vi "TLB Native Dynamic Events ver 0.26d.vi"() -> ()   [LabVIEW 2018] (continued)
                  tunnel: w1878 -> [w1884 w1890]
                  frame False {
                    n645 = for {
                      tunnel: string[] ["CLOSE CLAW", "START TIMER"] ("element") -> [w1887] mode=indexing
                      shift-right: [w1889] -> w1886
                      shift-left: w1884 -> [w1888]
                      n646 = Enqueue Element(queue=w1888, element=w1887) -> (queue out=w1889:refnum<queue>)  [unwired: 2 in, 2 out]
                    }
                  }
                  frame True {
                    n647 = for {
                      shift-right: [w1894] -> w1892
                      shift-left: w1890 -> [w1895]
                      tunnel: string[] ["READ STEPPER VALUES", "", ""] -> [w1893] mode=indexing
                      n648 = Enqueue Element(queue=w1895, element=w1893) -> (queue out=w1894:refnum<queue>)  [unwired: 2 in, 2 out]
                    }
                  }
                }
                n649 = Or(x=w1877, y=w1873) -> (x .or. y?=w1880:bool)
                n650 = Select(t=State_Type_Definitions,_for_0.26g_versions_and_later_2."True Stop" ("Enum"), s=w1873, f=State_Type_Definitions,_for_0.26g_versions_and_later_2."Task 8K: RAISE MY SWORD" ("Enum")) -> (s? t:f=w1875:T18)
                n651 = Select(t=w1875, s=w1880, f=State_Type_Definitions,_for_0.26g_versions_and_later_2."Task 8J: CLOSE CLAW" ("Enum")) -> (s? t:f=w1879:T18)
              }
              frame "Exit" {
                n652 = for {
                  shift-right: [w1902] -> w1899
                  shift-left: w1896 -> [w1903]
                  tunnel: string[] ["STOP", "RESET ENCODERS", "RESET YAW", "ARDUINO MODE 0"] -> [w1901] mode=indexing
                  n653 = Enqueue Element(queue=w1903, element=w1901) -> (queue out=w1902:refnum<queue>)  [unwired: 2 in, 2 out]
                }
              }
            }
          }
          frame 37 {
            # ">>> yStepper command>>>"
            # ">> Manual override >>"
            n654 = Dequeue Element(queue=w1914, timeout in ms (-1)=w1913, error in (no error)=w1915) -> (element=w1912:T10)  [unwired: 3 out]
            n655 = Equal?(x=w1911, y=u8 60) -> (x = y?=w1909:bool)
            n656 = case shown="\"Start Task 1\", Default" w1912 {
              tunnel: [w1925 State_Type_Definitions,_for_0.26g_versions_and_later_2."True Stop" ("Enum")] -> w1916
              tunnel: [w1928 w1945] -> w1917
              tunnel: [State_Type_Definitions,_for_0.26g_versions_and_later_2."Idle" ("Enum") State_Type_Definitions,_for_0.26g_versions_and_later_2."Shutdown" ("Enum")] -> w1918
              tunnel: w1909 -> [w1924 _]
              tunnel: w1908 -> [w1923 _]
              tunnel: w1907 -> [w1919 w1942]
              frame "Start Task 1", Default {
                # "Stays in Task 5_A until stepper reaches desired \nheight"
                # "T: Go back to idle, F: Continue with task\""
                # ">> Manual override >>"
                n657 = case shown="True" w1924 {
                  tunnel: [w1932 w1938] -> w1928
                  tunnel: w1919 -> [w1930 w1936]
                  frame False {
                    n658 = for {
                      tunnel: string[] ["Z STEPPER CAM HEIGHT", "READ STEPPER VALUES"] ("element") -> [w1933] mode=indexing
                      shift-right: [w1935] -> w1932
                      shift-left: w1930 -> [w1934]
                      n659 = Enqueue Element(queue=w1934, element=w1933) -> (queue out=w1935:refnum<queue>)  [unwired: 2 in, 2 out]
                    }
                  }
                  frame True {
                    n660 = for {
                      shift-right: [w1940] -> w1938
                      shift-left: w1936 -> [w1941]
                      tunnel: string[] ["CAM CLOSE", "DISPOSE CAM BUFFERS", "DISPOSE PROC BUFFERS", "RESET ENCODERS"] -> [w1939] mode=indexing
                      n661 = Enqueue Element(queue=w1941, element=w1939) -> (queue out=w1940:refnum<queue>)  [unwired: 2 in, 2 out]
                    }
                  }
                }
                n662 = Or(x=w1924, y=w1923) -> (x .or. y?=w1926:bool)
                n663 = Select(t=State_Type_Definitions,_for_0.26g_versions_and_later_2."True Stop" ("Enum"), s=w1923, f=State_Type_Definitions,_for_0.26g_versions_and_later_2."True Stop" ("Enum")) -> (s? t:f=w1920:T18)
                n664 = Select(t=w1920, s=w1926, f=State_Type_Definitions,_for_0.26g_versions_and_later_2."Task 8K: RAISE MY SWORD" ("Enum")) -> (s? t:f=w1925:T18)
              }
              frame "Exit" {
                n665 = for {
                  shift-right: [w1948] -> w1945
                  shift-left: w1942 -> [w1949]
                  tunnel: string[] ["STOP", "RESET ENCODERS", "RESET YAW", "ARDUINO MODE 0"] -> [w1947] mode=indexing
                  n666 = Enqueue Element(queue=w1949, element=w1947) -> (queue out=w1948:refnum<queue>)  [unwired: 2 in, 2 out]
                }
              }
            }
          }
          frame 38 {
            # ">>> Motor control cluster >>>"
            # ">> Stepper height reeached >>"
            # ">>> yStepper command>>>"
            # ">> Manual override >>"
            n667 = Dequeue Element(queue=w1961, timeout in ms (-1)=w1956, error in (no error)=w1960) -> (element=w1964:T10)  [unwired: 3 out]
            n668 = Equal?(x=w1958, y=u8 50) -> (x = y?=w1962:bool)
            n669 = case shown="\"Start Task 1\", Default" w1964 {
              tunnel: [w1975 State_Type_Definitions,_for_0.26g_versions_and_later_2."True Stop" ("Enum")] -> w1954
              tunnel: [w1973 w1990] -> w1953
              tunnel: w1957 -> [w1972 _]
              tunnel: w1959 -> [w1966 _]
              tunnel: [State_Type_Definitions,_for_0.26g_versions_and_later_2."Idle" ("Enum") State_Type_Definitions,_for_0.26g_versions_and_later_2."Shutdown" ("Enum")] -> w1955
              tunnel: w1962 -> [w1965 _]
              frame "Start Task 1", Default {
                # ">> WIill proceed to part ii if not manual override >>"
                # ">>If ENABLE or Trigger is set to true>>"
                n670 = Or(x=w1965, y=w1966) -> (x .or. y?=w1967:bool)
                n671 = case shown="False" w1965 {
                  tunnel: [w1978 w1984] -> w1973
                  tunnel: w1972 -> [w1977 w1983]
                  frame False {
                    n672 = for {
                      shift-right: [w1980] -> w1978
                      shift-left: w1977 -> [w1981]
                      tunnel: string[] ["Z STEPPER BOX HEIGHT", "READ STEPPER VALUES"] ("element") -> [w1979] mode=indexing
                      n673 = Enqueue Element(queue=w1981, element=w1979) -> (queue out=w1980:refnum<queue>)  [unwired: 2 in, 2 out]
                    }
                  }
                  frame True {
                    n674 = for {
                      shift-right: [w1986] -> w1984
                      shift-left: w1983 -> [w1987]
                      tunnel: string[] ["READ NAVX", "RESET FLAGS", "", "", "", ""] -> [w1985] mode=indexing
                      n675 = Enqueue Element(queue=w1987, element=w1985) -> (queue out=w1986:refnum<queue>)  [unwired: 2 in, 2 out]
                    }
                  }
                }
                n676 = Select(t=State_Type_Definitions,_for_0.26g_versions_and_later_2."True Stop" ("Enum"), s=w1966, f=State_Type_Definitions,_for_0.26g_versions_and_later_2."Task 9B: Rotate to Angle" ("Enum")) -> (s? t:f=w1969:T18)
                n677 = Select(t=w1969, s=w1967, f=State_Type_Definitions,_for_0.26g_versions_and_later_2."Task 9A: Raise Arm" ("Enum")) -> (s? t:f=w1975:T18)
              }
              frame "Exit" {
                n678 = for {
                  shift-right: [w1993] -> w1990
                  shift-left: _ -> [w1994]
                  tunnel: string[] ["STOP", "RESET ENCODERS", "RESET YAW", ""] -> [w1992] mode=indexing
                  n679 = Enqueue Element(queue=w1994, element=w1992) -> (queue out=w1993:refnum<queue>)  [unwired: 2 in, 2 out]
                }
              }
            }
          }
          frame 39 {
            # ">>> Motor control cluster >>>"
            # ">>> yStepper command>>>"
            n680 = Dequeue Element(queue=w2008, timeout in ms (-1)=w2007, error in (no error)=w2006) -> (element=w2010:T10)  [unwired: 3 out]
            n681 = In Range and Coerce(upper limit=65.0, x=w2000, lower limit=58.0) -> (In Range?=w1997:bool)  [unwired: 1 out]
            n682 = case shown="\"Start Task 1\", Default" w2010 {
              tunnel: w2001 -> [w2013 _]
              tunnel: [w2021 State_Type_Definitions,_for_0.26g_versions_and_later_2."True Stop" ("Enum")] -> w2003
              tunnel: w2009 -> [w2019 w2037]
              tunnel: [w2018 w2036] -> w2002
              tunnel: [State_Type_Definitions,_for_0.26g_versions_and_later_2."Idle" ("Enum") State_Type_Definitions,_for_0.26g_versions_and_later_2."Shutdown" ("Enum")] -> w2004
              tunnel: w1997 -> [w2011 _]
              frame "Start Task 1", Default {
                n683 = Or(x=w2011, y=w2013) -> (x .or. y?=w2012:bool)
                n684 = case shown="True" w2011 {
                  tunnel: w2019 -> [w2024 w2030]
                  tunnel: [w2023 w2028] -> w2018
                  frame False {
                    n685 = for {
                      shift-right: [w2026] -> w2023
                      shift-left: w2024 -> [w2027]
                      tunnel: string[] ["READ NAVX", "R-CW", ""] ("element") -> [w2025] mode=indexing
                      n686 = Enqueue Element(queue=w2027, element=w2025) -> (queue out=w2026:refnum<queue>)  [unwired: 2 in, 2 out]
                    }
                  }
                  frame True {
                    n687 = for {
                      shift-right: [w2032] -> w2028
                      shift-left: w2030 -> [w2033]
                      tunnel: string[] ["STOP", "RESET ENCODERS", "RESET YAW", "", ""] -> [w2031] mode=indexing
                      n688 = Enqueue Element(queue=w2033, element=w2031) -> (queue out=w2032:refnum<queue>)  [unwired: 2 in, 2 out]
                    }
                  }
                }
                n689 = Select(t=State_Type_Definitions,_for_0.26g_versions_and_later_2."True Stop" ("Enum"), s=w2013, f=State_Type_Definitions,_for_0.26g_versions_and_later_2."Task 9C: Detect Box") -> (s? t:f=w2015:T18)
                n690 = Select(t=w2015, s=w2012, f=State_Type_Definitions,_for_0.26g_versions_and_later_2."Task 9B: Rotate to Angle" ("Enum")) -> (s? t:f=w2021:T18)
              }
              frame "Exit" {
                n691 = for {
                  shift-right: [w2040] -> w2036
                  shift-left: w2037 -> [w2041]
                  tunnel: string[] ["STOP", "RESET ENCODERS", "RESET YAW", ""] -> [w2039] mode=indexing
                  n692 = Enqueue Element(queue=w2041, element=w2039) -> (queue out=w2040:refnum<queue>)  [unwired: 2 in, 2 out]
                }
              }
            }
          }
          frame 40 {
            # ">>> Motor control cluster >>>"
            # ">>Line Detected>>"
            # ">>Action Queue>>"
            # ">>> yStepper command>>>"
            n693 = Dequeue Element(queue=w2053, timeout in ms (-1)=w2052, error in (no error)=w2051) -> (element=w2054:T10)  [unwired: 3 out]
            n694 = case shown="\"Start Task 1\", Default" w2054 {
              tunnel: w2049 -> [w2055 _]
              tunnel: [w2065 State_Type_Definitions,_for_0.26g_versions_and_later_2."True Stop" ("Enum")] -> w2046
              tunnel: w2050 -> [w2063 w2081]
              tunnel: [w2062 w2080] -> w2045
              tunnel: [State_Type_Definitions,_for_0.26g_versions_and_later_2."Idle" ("Enum") State_Type_Definitions,_for_0.26g_versions_and_later_2."Shutdown" ("Enum")] -> w2048
              tunnel: w2043 -> [w2056 _]
              frame "Start Task 1", Default {
                n695 = Or(x=w2055, y=w2056) -> (x .or. y?=w2057:bool)
                n696 = case shown="True" w2056 {
                  tunnel: w2063 -> [w2068 w2074]
                  tunnel: [w2067 w2072] -> w2062
                  frame False {
                    n697 = for {
                      shift-right: [w2070] -> w2067
                      shift-left: w2068 -> [w2071]
                      tunnel: string[] ["READ IR", "READ LINE SENSOR", "FORWARD - IR ASSIST"] ("element") -> [w2069] mode=indexing
                      n698 = Enqueue Element(queue=w2071, element=w2069) -> (queue out=w2070:refnum<queue>)  [unwired: 2 in, 2 out]
                    }
                  }
                  frame True {
                    n699 = for {
                      shift-right: [w2076] -> w2072
                      shift-left: w2074 -> [w2077]
                      tunnel: string[] ["STOP", "RESET ENCODERS", "RESET YAW", "RESET FLAGS"] -> [w2075] mode=indexing
                      n700 = Enqueue Element(queue=w2077, element=w2075) -> (queue out=w2076:refnum<queue>)  [unwired: 2 in, 2 out]
                    }
                  }
                }
                n701 = Select(t=State_Type_Definitions,_for_0.26g_versions_and_later_2."True Stop" ("Enum"), s=w2055, f=State_Type_Definitions,_for_0.26g_versions_and_later_2."Task 9D: MOVE FORWARD") -> (s? t:f=w2059:T18)
                n702 = Select(t=w2059, s=w2057, f=State_Type_Definitions,_for_0.26g_versions_and_later_2."Task 9C: Detect Box" ("Enum")) -> (s? t:f=w2065:T18)
              }
              frame "Exit" {
                n703 = for {
                  shift-right: [w2084] -> w2080
                  shift-left: w2081 -> [w2085]
                  tunnel: string[] ["STOP", "RESET ENCODERS", "RESET YAW", ""] -> [w2083] mode=indexing
                  n704 = Enqueue Element(queue=w2085, element=w2083) -> (queue out=w2084:refnum<queue>)  [unwired: 2 in, 2 out]
                }
              }
            }
          }
          frame 41 {
            (unwired) 50.0 ("y")
            # ">> Item Selection Bias >>"
            # ">> Wall detected >>"
            # ">> Manual override >>"
            # ">>Table Detected>>"
            # ">>> Motor control cluster >>>"
            # ">>Table or wall detectected>>"
            # ">>Action Queue>>"
            # ">>> yStepper command>>>"
            n705 = Dequeue Element(queue=w2103, timeout in ms (-1)=w2102, error in (no error)=w2101) -> (element=w2104:T10)  [unwired: 3 out]
            n706 = Less Or Equal?(x=w2092, y=18.0) -> (x <= y?=w2087:bool)
            n707 = Less?(x=w2090, y=20.0) -> (x < y?=w2088:bool)
            n708 = Or(x=w2087, y=w2088) -> (x .or. y?=w2086:bool)
            n709 = case shown="\"Start Task 1\", Default" w2104 {
              tunnel: w2099 -> [w2105 _]
              tunnel: [w2115 State_Type_Definitions,_for_0.26g_versions_and_later_2."True Stop" ("Enum")] -> w2096
              tunnel: w2100 -> [w2113 w2131]
              tunnel: [w2112 w2130] -> w2095
              tunnel: [State_Type_Definitions,_for_0.26g_versions_and_later_2."Idle" ("Enum") State_Type_Definitions,_for_0.26g_versions_and_later_2."Shutdown" ("Enum")] -> w2098
              tunnel: w2086 -> [w2106 _]
              frame "Start Task 1", Default {
                n710 = Or(x=w2105, y=w2106) -> (x .or. y?=w2107:bool)
                n711 = case shown="True" w2106 {
                  tunnel: w2113 -> [w2118 w2124]
                  tunnel: [w2117 w2122] -> w2112
                  frame False {
                    n712 = for {
                      shift-right: [w2120] -> w2117
                      shift-left: w2118 -> [w2121]
                      tunnel: string[] ["READ IR", "FORWARD - IR ASSIST", ""] ("element") -> [w2119] mode=indexing
                      n713 = Enqueue Element(queue=w2121, element=w2119) -> (queue out=w2120:refnum<queue>)  [unwired: 2 in, 2 out]
                    }
                  }
                  frame True {
                    n714 = for {
                      shift-right: [w2126] -> w2122
                      shift-left: w2124 -> [w2127]
                      tunnel: string[] ["STOP", "RESET ENCODERS", "RESET YAW", "RESET FLAGS"] -> [w2125] mode=indexing
                      n715 = Enqueue Element(queue=w2127, element=w2125) -> (queue out=w2126:refnum<queue>)  [unwired: 2 in, 2 out]
                    }
                  }
                }
                n716 = Select(t=State_Type_Definitions,_for_0.26g_versions_and_later_2."True Stop" ("Enum"), s=w2105, f=State_Type_Definitions,_for_0.26g_versions_and_later_2."Task 9E: MOVE LEFT") -> (s? t:f=w2109:T18)
                n717 = Select(t=w2109, s=w2107, f=State_Type_Definitions,_for_0.26g_versions_and_later_2."Task 9D: MOVE FORWARD" ("Enum")) -> (s? t:f=w2115:T18)
              }
              frame "Exit" {
                n718 = for {
                  shift-right: [w2134] -> w2130
                  shift-left: w2131 -> [w2135]
                  tunnel: string[] ["STOP", "RESET ENCODERS", "RESET YAW", ""] -> [w2133] mode=indexing
                  n719 = Enqueue Element(queue=w2135, element=w2133) -> (queue out=w2134:refnum<queue>)  [unwired: 2 in, 2 out]
                }
              }
            }
          }
          frame 42 {
            # ">> Item Selection Bias >>"
            # ">> Line detected? >>"
            # ">> Manual override >>"
            # ">>> Motor control cluster >>>"
            # ">>Action Queue>>"
            # ">>> yStepper command>>>"
            n720 = Dequeue Element(queue=w2147, timeout in ms (-1)=w2146, error in (no error)=w2145) -> (element=w2148:T10)  [unwired: 3 out]
            n721 = case shown="\"Start Task 1\", Default" w2148 {
              tunnel: w2143 -> [w2149 _]
              tunnel: [w2159 State_Type_Definitions,_for_0.26g_versions_and_later_2."True Stop" ("Enum")] -> w2140
              tunnel: w2144 -> [w2157 w2175]
              tunnel: [w2156 w2174] -> w2139
              tunnel: [State_Type_Definitions,_for_0.26g_versions_and_later_2."Idle" ("Enum") State_Type_Definitions,_for_0.26g_versions_and_later_2."Shutdown" ("Enum")] -> w2142
              tunnel: w2136 -> [w2150 _]
              frame "Start Task 1", Default {
                n722 = Or(x=w2149, y=w2150) -> (x .or. y?=w2151:bool)
                n723 = case shown="True" w2150 {
                  tunnel: w2157 -> [w2162 w2168]
                  tunnel: [w2161 w2166] -> w2156
                  frame False {
                    n724 = for {
                      shift-right: [w2164] -> w2161
                      shift-left: w2162 -> [w2165]
                      tunnel: string[] ["LEFT", "READ NAVX", "READ LINE SENSOR", ""] ("element") -> [w2163] mode=indexing
                      n725 = Enqueue Element(queue=w2165, element=w2163) -> (queue out=w2164:refnum<queue>)  [unwired: 2 in, 2 out]
                    }
                  }
                  frame True {
                    n726 = for {
                      shift-right: [w2170] -> w2166
                      shift-left: w2168 -> [w2171]
                      tunnel: string[] ["STOP", "RESET ENCODERS", "RESET YAW", "BOX COLOUR", "", ""] -> [w2169] mode=indexing
                      n727 = Enqueue Element(queue=w2171, element=w2169) -> (queue out=w2170:refnum<queue>)  [unwired: 2 in, 2 out]
                    }
                  }
                }
                n728 = Select(t=State_Type_Definitions,_for_0.26g_versions_and_later_2."True Stop" ("Enum"), s=w2149, f=State_Type_Definitions,_for_0.26d_versions_and_later."Task 9F: Detect Box Colour") -> (s? t:f=w2153:u16)
                n729 = Select(t=w2153, s=w2151, f=State_Type_Definitions,_for_0.26g_versions_and_later_2."Task 9E: MOVE LEFT" ("Enum")) -> (s? t:f=w2159:u16)
              }
              frame "Exit" {
                n730 = for {
                  shift-right: [w2178] -> w2174
                  shift-left: w2175 -> [w2179]
                  tunnel: string[] ["STOP", "RESET ENCODERS", "RESET YAW", ""] -> [w2177] mode=indexing
                  n731 = Enqueue Element(queue=w2179, element=w2177) -> (queue out=w2178:refnum<queue>)  [unwired: 2 in, 2 out]
                }
              }
            }
          }
          frame 43 {
            # ">>> Motor control cluster >>>"
            # ">>Colour detection >>"
            # ">>> yStepper command>>>"
            # ">> Manual override >>"
            n732 = Dequeue Element(queue=w2192, timeout in ms (-1)=w2190, error in (no error)=w2191) -> (element=w2185:T10)  [unwired: 3 out]
            n733 = case shown="\"Start Task 1\", Default" w2185 {
              tunnel: [w2203 State_Type_Definitions,_for_0.26g_versions_and_later_2."True Stop" ("Enum")] -> w2181
              tunnel: [w2201 w2218] -> w2182
              tunnel: w2184 -> [w2200 _]
              tunnel: w2186 -> [w2194 _]
              tunnel: [State_Type_Definitions,_for_0.26g_versions_and_later_2."Idle" ("Enum") State_Type_Definitions,_for_0.26g_versions_and_later_2."Shutdown" ("Enum")] -> w2180
              tunnel: w2183 -> [w2193 _]
              frame "Start Task 1", Default {
                # ">> WIill proceed to part ii if not manual override >>"
                # ">>If ENABLE or Trigger is set to true>>"
                n734 = Or(x=w2193, y=w2194) -> (x .or. y?=w2195:bool)
                n735 = case shown="True" w2193 {
                  tunnel: [w2206 w2212] -> w2201
                  tunnel: w2200 -> [w2205 w2211]
                  frame False {
                    n736 = for {
                      shift-right: [w2208] -> w2206
                      shift-left: w2205 -> [w2209]
                      tunnel: string[] ["", ""] ("element") -> [w2207] mode=indexing
                      n737 = Enqueue Element(queue=w2209, element=w2207) -> (queue out=w2208:refnum<queue>)  [unwired: 2 in, 2 out]
                    }
                  }
                  frame True {
                    n738 = for {
                      shift-right: [w2214] -> w2212
                      shift-left: w2211 -> [w2215]
                      tunnel: string[] ["RESET ENCODER", "RESET FLAGS", "RESET YAW", "", "", ""] -> [w2213] mode=indexing
                      n739 = Enqueue Element(queue=w2215, element=w2213) -> (queue out=w2214:refnum<queue>)  [unwired: 2 in, 2 out]
                    }
                  }
                }
                n740 = Select(t=State_Type_Definitions,_for_0.26g_versions_and_later_2."True Stop" ("Enum"), s=w2194, f=State_Type_Definitions,_for_0.26g_versions_and_later_2."True Stop" ("Enum")) -> (s? t:f=w2197:T18)
                n741 = Select(t=w2197, s=w2195, f=State_Type_Definitions,_for_0.26d_versions_and_later."Task 9F: Detect Box Colour" ("Enum")) -> (s? t:f=w2203:u16)
              }
              frame "Exit" {
                n742 = for {
                  shift-right: [w2221] -> w2218
                  shift-left: _ -> [w2222]
                  tunnel: string[] ["STOP", "RESET ENCODERS", "RESET YAW", ""] -> [w2220] mode=indexing
                  n743 = Enqueue Element(queue=w2222, element=w2220) -> (queue out=w2221:refnum<queue>)  [unwired: 2 in, 2 out]
                }
              }
            }
          }
          frame 44 {
            # ">>> Motor control cluster >>>"
            # ">>> yStepper command>>>"
            n744 = Dequeue Element(queue=w2234, timeout in ms (-1)=w2233, error in (no error)=w2232) -> (element=w2239:T10)  [unwired: 3 out]
            n745 = Greater?(x=w2224, y=50.0) -> (0:w2227:bool)
            n746 = And(x=w2225, y=w2227) -> (x .and. y?=w2223:bool)
            n747 = case shown="\"Start Task 1\", Default" w2239 {
              tunnel: w2223 -> [w2242 _]
              tunnel: [w2249 State_Type_Definitions,_for_0.26g_versions_and_later_2."True Stop" ("Enum")] -> w2238
              tunnel: w2231 -> [w2241 _]
              tunnel: w2235 -> [w2248 w2265]
              tunnel: [w2247 w2266] -> w2237
              tunnel: [State_Type_Definitions,_for_0.26g_versions_and_later_2."Idle" ("Enum") State_Type_Definitions,_for_0.26g_versions_and_later_2."Shutdown" ("Enum")] -> w2236
              frame "Start Task 1", Default {
                n748 = case shown="True" w2242 {
                  tunnel: w2248 -> [w2252 w2259]
                  tunnel: [w2253 w2258] -> w2247
                  frame False {
                    n749 = for {
                      tunnel: string[] ["READ LINE SENSOR", "READ NAVX", "RIGHT", "READ ENCODERS"] ("element") -> [w2254] mode=indexing
                      shift-right: [w2256] -> w2253
                      shift-left: w2252 -> [w2255]
                      n750 = Enqueue Element(queue=w2255, element=w2254) -> (queue out=w2256:refnum<queue>)  [unwired: 2 in, 2 out]
                    }
                  }
                  frame True {
                    n751 = for {
                      shift-right: [w2261] -> w2258
                      shift-left: w2259 -> [w2262]
                      tunnel: string[] ["RESET ENCODERS", "RESET YAW", "RESET FLAGS", "Box Colour", ""] -> [w2260] mode=indexing
                      n752 = Enqueue Element(queue=w2262, element=w2260) -> (queue out=w2261:refnum<queue>)  [unwired: 2 in, 2 out]
                    }
                  }
                }
                n753 = Or(x=w2242, y=w2241) -> (x .or. y?=w2240:bool)
                n754 = Select(t=State_Type_Definitions,_for_0.26g_versions_and_later_2."True Stop" ("Enum"), s=w2241, f=State_Type_Definitions,_for_0.26d_versions_and_later."Task 9H: Box Detection" ("Enum")) -> (s? t:f=w2243:u16)
                n755 = Select(t=w2243, s=w2240, f=State_Type_Definitions,_for_0.26g_versions_and_later_2."Task 9G: MOVE RIGHT" ("Enum")) -> (s? t:f=w2249:u16)
              }
              frame "Exit" {
                n756 = for {
                  shift-right: [w2269] -> w2266
                  shift-left: w2265 -> [w2270]
                  tunnel: string[] ["STOP", "RESET ENCODERS", "RESET YAW", "ARDUINO MODE 0"] -> [w2268] mode=indexing
                  n757 = Enqueue Element(queue=w2270, element=w2268) -> (queue out=w2269:refnum<queue>)  [unwired: 2 in, 2 out]
                }
              }
            }
          }
          frame 45 {
            # ">> Item Selection Bias >>"
            # ">>> Motor control cluster >>>"
            # ">>> yStepper command>>>"
            n758 = Dequeue Element(queue=w2276, timeout in ms (-1)=w2277, error in (no error)=w2278) -> (element=w2280:T10)  [unwired: 3 out]
            n759 = case shown="\"Start Task 1\", Default" w2280 {
              tunnel: w2271 -> [w2286 _]
              tunnel: [w2293 State_Type_Definitions,_for_0.26g_versions_and_later_2."True Stop" ("Enum")] -> w2273
              tunnel: w2279 -> [w2285 _]
              tunnel: w2275 -> [w2292 w2309]
              tunnel: [w2291 w2310] -> w2274
              tunnel: [State_Type_Definitions,_for_0.26g_versions_and_later_2."Idle" ("Enum") State_Type_Definitions,_for_0.26g_versions_and_later_2."Shutdown" ("Enum")] -> w2272
              frame "Start Task 1", Default {
                n760 = case shown="False" w2286 {
                  tunnel: w2292 -> [w2296 w2303]
                  tunnel: [w2297 w2302] -> w2291
                  frame False {
                    n761 = for {
                      tunnel: string[] ["Box Colour", "", "", ""] ("element") -> [w2298] mode=indexing
                      shift-right: [w2300] -> w2297
                      shift-left: w2296 -> [w2299]
                      n762 = Enqueue Element(queue=w2299, element=w2298) -> (queue out=w2300:refnum<queue>)  [unwired: 2 in, 2 out]
                    }
                  }
                  frame True {
                    n763 = for {
                      shift-right: [w2305] -> w2302
                      shift-left: w2303 -> [w2306]
                      tunnel: string[] ["DISPOSE BUFFERS", "", "", "", "", ""] -> [w2304] mode=indexing
                      n764 = Enqueue Element(queue=w2306, element=w2304) -> (queue out=w2305:refnum<queue>)  [unwired: 2 in, 2 out]
                    }
                  }
                }
                n765 = Or(x=w2286, y=w2285) -> (x .or. y?=w2284:bool)
                n766 = Select(t=State_Type_Definitions,_for_0.26g_versions_and_later_2."True Stop" ("Enum"), s=w2285, f=State_Type_Definitions,_for_0.26g_versions_and_later_2."True Stop" ("Enum")) -> (s? t:f=w2287:T18)
                n767 = Select(t=w2287, s=w2284, f=State_Type_Definitions,_for_0.26d_versions_and_later."Task 9H: Box Detection" ("Enum")) -> (s? t:f=w2293:u16)
              }
              frame "Exit" {
                n768 = for {
                  shift-right: [w2313] -> w2310
                  shift-left: w2309 -> [w2314]
                  tunnel: string[] ["STOP", "RESET ENCODERS", "RESET YAW", "ARDUINO MODE 0"] -> [w2312] mode=indexing
                  n769 = Enqueue Element(queue=w2314, element=w2312) -> (queue out=w2313:refnum<queue>)  [unwired: 2 in, 2 out]
                }
              }
            }
          }
          frame 46 {
            # ">> Item Selection Bias >>"
            n770 = Dequeue Element(queue=w2316, timeout in ms (-1)=w2317, error in (no error)=w2318) -> (element=w2324:T10)  [unwired: 3 out]
            n771 = case shown="\"Start Task 1\", Default" w2324 {
              tunnel: w2315 -> [w2330 _]
              tunnel: [w2337 State_Type_Definitions,_for_0.26g_versions_and_later_2."True Stop" ("Enum")] -> w2321
              tunnel: w2319 -> [w2329 _]
              tunnel: w2323 -> [w2336 w2353]
              tunnel: [w2335 w2354] -> w2322
              tunnel: [State_Type_Definitions,_for_0.26g_versions_and_later_2."Idle" ("Enum") State_Type_Definitions,_for_0.26g_versions_and_later_2."Shutdown" ("Enum")] -> w2320
              frame "Start Task 1", Default {
                n772 = case shown="True" w2330 {
                  tunnel: w2336 -> [w2340 w2347]
                  tunnel: [w2341 w2346] -> w2335
                  frame False {
                    n773 = for {
                      tunnel: string[] ["START TIMER", "CAM ACQ", ""] ("element") -> [w2342] mode=indexing
                      shift-right: [w2344] -> w2341
                      shift-left: w2340 -> [w2343]
                      n774 = Enqueue Element(queue=w2343, element=w2342) -> (queue out=w2344:refnum<queue>)  [unwired: 2 in, 2 out]
                    }
                  }
                  frame True {
                    n775 = for {
                      shift-right: [w2349] -> w2346
                      shift-left: w2347 -> [w2350]
                      tunnel: string[] ["CLOSE CAM", "SET TIMER 5", "", "", "", ""] -> [w2348] mode=indexing
                      n776 = Enqueue Element(queue=w2350, element=w2348) -> (queue out=w2349:refnum<queue>)  [unwired: 2 in, 2 out]
                    }
                  }
                }
                n777 = Or(x=w2330, y=w2329) -> (x .or. y?=w2328:bool)
                n778 = Select(t=State_Type_Definitions,_for_0.26g_versions_and_later_2."True Stop" ("Enum"), s=w2329, f=State_Type_Definitions,_for_0.26d_versions_and_later."Task 9J: PROCESS COLOUR" ("Enum")) -> (s? t:f=w2331:u16)
                n779 = Select(t=w2331, s=w2328, f=State_Type_Definitions,_for_0.26d_versions_and_later."Task 9I: SCAN IMAGE" ("Enum")) -> (s? t:f=w2337:u16)
              }
              frame "Exit" {
                n780 = for {
                  shift-right: [w2357] -> w2354
                  shift-left: w2353 -> [w2358]
                  tunnel: string[] ["STOP", "RESET ENCODERS", "RESET YAW", "ARDUINO MODE 0"] -> [w2356] mode=indexing
                  n781 = Enqueue Element(queue=w2358, element=w2356) -> (queue out=w2357:refnum<queue>)  [unwired: 2 in, 2 out]
                }
              }
            }
          }
          frame 47 {
            # ">> Item Selection Bias >>"
            n782 = Dequeue Element(queue=w2364, timeout in ms (-1)=w2365, error in (no error)=w2366) -> (element=w2368:T10)  [unwired: 3 out]
            n783 = case shown="\"Start Task 1\", Default" w2368 {
              tunnel: w2359 -> [w2374 _]
              tunnel: [w2381 State_Type_Definitions,_for_0.26g_versions_and_later_2."True Stop" ("Enum")] -> w2362
              tunnel: w2367 -> [w2373 _]
              tunnel: w2363 -> [w2380 w2397]
              tunnel: [w2379 w2398] -> w2361
              tunnel: [State_Type_Definitions,_for_0.26g_versions_and_later_2."Idle" ("Enum") State_Type_Definitions,_for_0.26g_versions_and_later_2."Shutdown" ("Enum")] -> w2360
              frame "Start Task 1", Default {
                n784 = case shown="True" w2374 {
                  tunnel: w2380 -> [w2384 w2391]
                  tunnel: [w2385 w2390] -> w2379
                  frame False {
                    n785 = for {
                      tunnel: string[] ["START TIMER", "COLOUR PROCESSING", ""] ("element") -> [w2386] mode=indexing
                      shift-right: [w2388] -> w2385
                      shift-left: w2384 -> [w2387]
                      n786 = Enqueue Element(queue=w2387, element=w2386) -> (queue out=w2388:refnum<queue>)  [unwired: 2 in, 2 out]
                    }
                  }
                  frame True {
                    n787 = for {
                      shift-right: [w2393] -> w2390
                      shift-left: w2391 -> [w2394]
                      tunnel: string[] ["CLOSE CAM", "DISPOSE BUFFERS", "RESET ENCODERS", "RESET YAW", "RESET FLAGS", ""] -> [w2392] mode=indexing
                      n788 = Enqueue Element(queue=w2394, element=w2392) -> (queue out=w2393:refnum<queue>)  [unwired: 2 in, 2 out]
                    }
                  }
                }
                n789 = Or(x=w2374, y=w2373) -> (x .or. y?=w2372:bool)
                n790 = Select(t=State_Type_Definitions,_for_0.26g_versions_and_later_2."True Stop" ("Enum"), s=w2373, f=State_Type_Definitions,_for_0.26g_versions_and_later_2."True Stop" ("Enum")) -> (s? t:f=w2375:T18)
                n791 = Select(t=w2375, s=w2372, f=State_Type_Definitions,_for_0.26d_versions_and_later."Task 9J: PROCESS COLOUR" ("Enum")) -> (s? t:f=w2381:u16)
              }
              frame "Exit" {
                n792 = for {
                  shift-right: [w2401] -> w2398
                  shift-left: w2397 -> [w2402]
                  tunnel: string[] ["STOP", "RESET ENCODERS", "RESET YAW", "ARDUINO MODE 0"] -> [w2400] mode=indexing
                  n793 = Enqueue Element(queue=w2402, element=w2400) -> (queue out=w2401:refnum<queue>)  [unwired: 2 in, 2 out]
                }
              }
            }
          }
          frame 48 {
            # ">>> Motor control cluster >>>"
            # ">>> yStepper command>>>"
            # ">> Item Selection Bias >>"
            n794 = Less?(x=w2406, y=-38.0) -> (x < y?=w2404:bool)
            n795 = Dequeue Element(queue=w2412, timeout in ms (-1)=w2411, error in (no error)=w2410) -> (element=w2414:T10)  [unwired: 3 out]
            n796 = case shown="\"Start Task 1\", Default" w2414 {
              tunnel: w2404 -> [w2420 _]
              tunnel: [w2427 State_Type_Definitions,_for_0.26g_versions_and_later_2."True Stop" ("Enum")] -> w2408
              tunnel: w2409 -> [w2419 _]
              tunnel: w2413 -> [w2426 w2443]
              tunnel: [w2425 w2444] -> w2403
              tunnel: [State_Type_Definitions,_for_0.26g_versions_and_later_2."Idle" ("Enum") State_Type_Definitions,_for_0.26g_versions_and_later_2."Shutdown" ("Enum")] -> w2407
              frame "Start Task 1", Default {
                n797 = case shown="True" w2420 {
                  tunnel: w2426 -> [w2430 w2437]
                  tunnel: [w2431 w2436] -> w2425
                  frame False {
                    n798 = for {
                      tunnel: string[] ["READ ENCODERS", "R-CW"] ("element") -> [w2432] mode=indexing
                      shift-right: [w2434] -> w2431
                      shift-left: w2430 -> [w2433]
                      n799 = Enqueue Element(queue=w2433, element=w2432) -> (queue out=w2434:refnum<queue>)  [unwired: 2 in, 2 out]
                    }
                  }
                  frame True {
                    n800 = for {
                      shift-right: [w2439] -> w2436
                      shift-left: w2437 -> [w2440]
                      tunnel: string[] ["STOP", "RESET ENCODERS", "RESET FLAGS", "RESET YAW", "READ IR", "ARDUINO - ULTRASONIC"] -> [w2438] mode=indexing
                      n801 = Enqueue Element(queue=w2440, element=w2438) -> (queue out=w2439:refnum<queue>)  [unwired: 2 in, 2 out]
                    }
                  }
                }
                n802 = Or(x=w2420, y=w2419) -> (x .or. y?=w2418:bool)
                n803 = Select(t=State_Type_Definitions,_for_0.26g_versions_and_later_2."True Stop" ("Enum"), s=w2419, f=State_Type_Definitions,_for_0.26d_versions_and_later."Task 9L: MOVE FORWARD" ("Enum")) -> (s? t:f=w2421:u16)
                n804 = Select(t=w2421, s=w2418, f=State_Type_Definitions,_for_0.26d_versions_and_later."Task 9K: ROTATE 90 CW" ("Enum")) -> (s? t:f=w2427:u16)
              }
              frame "Exit" {
                n805 = for {
                  shift-right: [w2447] -> w2444
                  shift-left: w2443 -> [w2448]
                  tunnel: string[] ["STOP", "RESET ENCODERS", "RESET YAW", "ARDUINO MODE 0"] -> [w2446] mode=indexing
                  n806 = Enqueue Element(queue=w2448, element=w2446) -> (queue out=w2447:refnum<queue>)  [unwired: 2 in, 2 out]
                }
              }
            }
          }
          frame 49 {
            w2461 = u8 50 ("y")
            # ">>> Motor control cluster >>>"
            # ">>> yStepper command>>>"
            # ">> Item Selection Bias >>"
            n807 = Less?(x=w2463, y=w2461) -> (x < y?=w2456:bool)
            n808 = Dequeue Element(queue=w2467, timeout in ms (-1)=w2466, error in (no error)=w2465) -> (element=w2471:T10)  [unwired: 3 out]
            n809 = Less?(x=w2462, y=w2461) -> (x < y?=w2457:bool)
            n810 = And(x=w2457, y=w2456) -> (x .and. y?=w2449:bool)
            n811 = Less Or Equal?(x=w2460, y=15.0) -> (x <= y?=w2455:bool)
            n812 = Greater?(x=w2454, y=100.0) -> (0:w2453:bool)
            n813 = Or(x=w2455, y=w2449) -> (x .or. y?=w2451:bool)
            n814 = And(x=w2453, y=w2451) -> (x .and. y?=w2452:bool)
            n815 = case shown="\"Start Task 1\", Default" w2471 {
              tunnel: w2452 -> [w2477 _]
              tunnel: [w2484 State_Type_Definitions,_for_0.26g_versions_and_later_2."True Stop" ("Enum")] -> w2469
              tunnel: w2464 -> [w2476 _]
              tunnel: w2468 -> [w2483 w2500]
              tunnel: [w2482 w2501] -> w2458
              tunnel: [State_Type_Definitions,_for_0.26g_versions_and_later_2."Idle" ("Enum") State_Type_Definitions,_for_0.26g_versions_and_later_2."Shutdown" ("Enum")] -> w2470
              frame "Start Task 1", Default {
                n816 = case shown="True" w2477 {
                  tunnel: w2483 -> [w2487 w2494]
                  tunnel: [w2488 w2493] -> w2482
                  frame False {
                    n817 = for {
                      tunnel: string[] ["READ IR", "FORWARD", "READ NAVX", "READ ENCODERS"] ("element") -> [w2489] mode=indexing
                      shift-right: [w2491] -> w2488
                      shift-left: w2487 -> [w2490]
                      n818 = Enqueue Element(queue=w2490, element=w2489) -> (queue out=w2491:refnum<queue>)  [unwired: 2 in, 2 out]
                    }
                  }
                  frame True {
                    n819 = for {
                      shift-right: [w2496] -> w2493
                      shift-left: w2494 -> [w2497]
                      tunnel: string[] ["STOP", "RESET ENCODERS", "RESET FLAGS", "RESET YAW", "", ""] -> [w2495] mode=indexing
                      n820 = Enqueue Element(queue=w2497, element=w2495) -> (queue out=w2496:refnum<queue>)  [unwired: 2 in, 2 out]
                    }
                  }
                }
                n821 = Or(x=w2477, y=w2476) -> (x .or. y?=w2475:bool)
                n822 = Select(t=State_Type_Definitions,_for_0.26g_versions_and_later_2."True Stop" ("Enum"), s=w2476, f=State_Type_Definitions,_for_0.26g_versions_and_later_2."True Stop" ("Enum")) -> (s? t:f=w2478:T18)
                n823 = Select(t=w2478, s=w2475, f=State_Type_Definitions,_for_0.26d_versions_and_later."Task 9L: MOVE FORWARD" ("Enum")) -> (s? t:f=w2484:u16)
              }
              frame "Exit" {
                n824 = for {
                  shift-right: [w2504] -> w2501
                  shift-left: w2500 -> [w2505]
                  tunnel: string[] ["STOP", "RESET ENCODERS", "RESET YAW", "ARDUINO MODE 0"] -> [w2503] mode=indexing
                  n825 = Enqueue Element(queue=w2505, element=w2503) -> (queue out=w2504:refnum<queue>)  [unwired: 2 in, 2 out]
                }
              }
            }
          }
          frame 50 {
            # ">> Item Selection Bias >>"
            n826 = Dequeue Element(queue=w2510, timeout in ms (-1)=w2509, error in (no error)=w2508) -> (element=w2515:T10)  [unwired: 3 out]
            n827 = case shown="\"Start Task 1\", Default" w2515 {
              tunnel: w2506 -> [w2521 _]
              tunnel: [w2528 State_Type_Definitions,_for_0.26g_versions_and_later_2."True Stop" ("Enum")] -> w2513
              tunnel: w2507 -> [w2520 _]
              tunnel: w2511 -> [w2527 w2544]
              tunnel: [w2526 w2545] -> w2512
              tunnel: [State_Type_Definitions,_for_0.26g_versions_and_later_2."Idle" ("Enum") State_Type_Definitions,_for_0.26g_versions_and_later_2."Shutdown" ("Enum")] -> w2514
              frame "Start Task 1", Default {
                n828 = case shown="False" w2521 {
                  tunnel: w2527 -> [w2531 w2538]
                  tunnel: [w2532 w2537] -> w2526
                  frame False {
                    n829 = for {
                      tunnel: string[] ["READ LINE SENSOR", "READ NAVX", "RIGHT", "READ ENCODERS"] ("element") -> [w2533] mode=indexing
                      shift-right: [w2535] -> w2532
                      shift-left: w2531 -> [w2534]
                      n830 = Enqueue Element(queue=w2534, element=w2533) -> (queue out=w2535:refnum<queue>)  [unwired: 2 in, 2 out]
                    }
                  }
                  frame True {
                    n831 = for {
                      shift-right: [w2540] -> w2537
                      shift-left: w2538 -> [w2541]
                      tunnel: string[] ["STOP", "RESET ENCODERS", "RESET YAW", "OPEN LIFE CAM", "SET TIMER 2", "RESET FLAGS"] -> [w2539] mode=indexing
                      n832 = Enqueue Element(queue=w2541, element=w2539) -> (queue out=w2540:refnum<queue>)  [unwired: 2 in, 2 out]
                    }
                  }
                }
                n833 = Or(x=w2521, y=w2520) -> (x .or. y?=w2519:bool)
                n834 = Select(t=State_Type_Definitions,_for_0.26g_versions_and_later_2."True Stop" ("Enum"), s=w2520, f=State_Type_Definitions,_for_0.26d_versions_and_later."Task 9N: SCAN IMAGE" ("Enum")) -> (s? t:f=w2522:u16)
                n835 = Select(t=w2522, s=w2519, f=State_Type_Definitions,_for_0.26g_versions_and_later_2."Task 9M: MOVE RIGHT" ("Enum")) -> (s? t:f=w2528:u16)
              }
              frame "Exit" {
                n836 = for {
                  shift-right: [w2548] -> w2545
                  shift-left: w2544 -> [w2549]
                  tunnel: string[] ["STOP", "RESET ENCODERS", "RESET YAW", "ARDUINO MODE 0"] -> [w2547] mode=indexing
                  n837 = Enqueue Element(queue=w2549, element=w2547) -> (queue out=w2548:refnum<queue>)  [unwired: 2 in, 2 out]
                }
              }
            }
          }
          frame 51 {
            # ">> Manual override >>"
            n838 = Dequeue Element(queue=w2558, timeout in ms (-1)=w2557, error in (no error)=w2556) -> (element=w2559:T10)  [unwired: 3 out]
            n839 = case shown="\"Start Task 1\", Default" w2559 {
              tunnel: [w2573 State_Type_Definitions,_for_0.26g_versions_and_later_2."True Stop" ("Enum")] -> w2551
              tunnel: [w2571 w2589] -> w2550
              tunnel: w2554 -> [w2570 w2586]
              tunnel: w2555 -> [w2564 _]
              tunnel: [State_Type_Definitions,_for_0.26g_versions_and_later_2."Idle" ("Enum") State_Type_Definitions,_for_0.26g_versions_and_later_2."Shutdown" ("Enum")] -> w2552
              tunnel: w2553 -> [w2563 _]
              frame "Start Task 1", Default {
                # ">> WIill proceed to part ii if not manual override >>"
                # ">>If ENABLE or Trigger is set to true>>"
                n840 = Or(x=w2563, y=w2564) -> (x .or. y?=w2565:bool)
                n841 = case shown="False" w2563 {
                  tunnel: [w2576 w2582] -> w2571
                  tunnel: w2570 -> [w2575 w2581]
                  frame False {
                    n842 = for {
                      shift-right: [w2578] -> w2576
                      shift-left: w2575 -> [w2579]
                      tunnel: string[] ["CAM ACQ", "START TIMER"] ("element") -> [w2577] mode=indexing
                      n843 = Enqueue Element(queue=w2579, element=w2577) -> (queue out=w2578:refnum<queue>)  [unwired: 2 in, 2 out]
                    }
                  }
                  frame True {
                    n844 = for {
                      shift-right: [w2584] -> w2582
                      shift-left: w2581 -> [w2585]
                      tunnel: string[] ["CLOSE CAM", "SET TIMER 5", "", "", "", ""] -> [w2583] mode=indexing
                      n845 = Enqueue Element(queue=w2585, element=w2583) -> (queue out=w2584:refnum<queue>)  [unwired: 2 in, 2 out]
                    }
                  }
                }
                n846 = Select(t=State_Type_Definitions,_for_0.26g_versions_and_later_2."True Stop" ("Enum"), s=w2564, f=State_Type_Definitions,_for_0.26d_versions_and_later."Task 9O: PROCESS COLOUR" ("Enum")) -> (s? t:f=w2567:u16)
                n847 = Select(t=w2567, s=w2565, f=State_Type_Definitions,_for_0.26d_versions_and_later."Task 9N: SCAN IMAGE" ("Enum")) -> (s? t:f=w2573:u16)
              }
              frame "Exit" {
                n848 = for {
                  shift-right: [w2592] -> w2589
                  shift-left: w2586 -> [w2593]
                  tunnel: string[] ["STOP", "RESET ENCODERS", "RESET YAW", ""] -> [w2591] mode=indexing
                  n849 = Enqueue Element(queue=w2593, element=w2591) -> (queue out=w2592:refnum<queue>)  [unwired: 2 in, 2 out]
                }
              }
            }
          }
          frame 52 {
            # ">> Item Selection Bias >>"
            n850 = Dequeue Element(queue=w2601, timeout in ms (-1)=w2600, error in (no error)=w2599) -> (element=w2603:T10)  [unwired: 3 out]
            n851 = case shown="\"Start Task 1\", Default" w2603 {
              tunnel: w2594 -> [w2609 _]
              tunnel: [w2616 State_Type_Definitions,_for_0.26g_versions_and_later_2."True Stop" ("Enum")] -> w2597
              tunnel: w2598 -> [w2608 _]
              tunnel: w2602 -> [w2615 w2632]
              tunnel: [w2614 w2633] -> w2596
              tunnel: [State_Type_Definitions,_for_0.26g_versions_and_later_2."Idle" ("Enum") State_Type_Definitions,_for_0.26g_versions_and_later_2."Shutdown" ("Enum")] -> w2595
              frame "Start Task 1", Default {
                n852 = case shown="False" w2609 {
                  tunnel: w2615 -> [w2619 w2626]
                  tunnel: [w2620 w2625] -> w2614
                  frame False {
                    n853 = for {
                      tunnel: string[] ["START TIMER", "COLOUR PROCESSING", ""] ("element") -> [w2621] mode=indexing
                      shift-right: [w2623] -> w2620
                      shift-left: w2619 -> [w2622]
                      n854 = Enqueue Element(queue=w2622, element=w2621) -> (queue out=w2623:refnum<queue>)  [unwired: 2 in, 2 out]
                    }
                  }
                  frame True {
                    n855 = for {
                      shift-right: [w2628] -> w2625
                      shift-left: w2626 -> [w2629]
                      tunnel: string[] ["CLOSE CAM", "DISPOSE BUFFERS", "RESET ENCODERS", "RESET YAW", "RESET FLAGS", ""] -> [w2627] mode=indexing
                      n856 = Enqueue Element(queue=w2629, element=w2627) -> (queue out=w2628:refnum<queue>)  [unwired: 2 in, 2 out]
                    }
                  }
                }
                n857 = Or(x=w2609, y=w2608) -> (x .or. y?=w2607:bool)
                n858 = Select(t=State_Type_Definitions,_for_0.26g_versions_and_later_2."True Stop" ("Enum"), s=w2608, f=State_Type_Definitions,_for_0.26d_versions_and_later."Task 9P: MOVE RIGHT" ("Enum")) -> (s? t:f=w2610:u16)
                n859 = Select(t=w2610, s=w2607, f=State_Type_Definitions,_for_0.26d_versions_and_later."Task 9O: PROCESS COLOUR" ("Enum")) -> (s? t:f=w2616:u16)
              }
              frame "Exit" {
                n860 = for {
                  shift-right: [w2636] -> w2633
                  shift-left: w2632 -> [w2637]
                  tunnel: string[] ["STOP", "RESET ENCODERS", "RESET YAW", "ARDUINO MODE 0"] -> [w2635] mode=indexing
                  n861 = Enqueue Element(queue=w2637, element=w2635) -> (queue out=w2636:refnum<queue>)  [unwired: 2 in, 2 out]
                }
              }
            }
          }
          frame 53 {
            # ">> Item Selection Bias >>"
            n862 = Dequeue Element(queue=w2643, timeout in ms (-1)=w2642, error in (no error)=w2641) -> (element=w2651:T10)  [unwired: 3 out]
            n863 = Greater?(x=w2639, y=50.0) -> (0:w2649:bool)
            n864 = And(x=w2638, y=w2649) -> (x .and. y?=w2650:bool)
            n865 = case shown="\"Start Task 1\", Default" w2651 {
              tunnel: w2650 -> [w2657 _]
              tunnel: [w2664 State_Type_Definitions,_for_0.26g_versions_and_later_2."True Stop" ("Enum")] -> w2646
              tunnel: w2640 -> [w2656 _]
              tunnel: w2644 -> [w2663 w2680]
              tunnel: [w2662 w2681] -> w2645
              tunnel: [State_Type_Definitions,_for_0.26g_versions_and_later_2."Idle" ("Enum") State_Type_Definitions,_for_0.26g_versions_and_later_2."Shutdown" ("Enum")] -> w2647
              frame "Start Task 1", Default {
                n866 = case shown="False" w2657 {
                  tunnel: w2663 -> [w2667 w2674]
                  tunnel: [w2668 w2673] -> w2662
                  frame False {
                    n867 = for {
                      tunnel: string[] ["READ LINE SENSOR", "READ NAVX", "RIGHT", "READ ENCODERS"] ("element") -> [w2669] mode=indexing
                      shift-right: [w2671] -> w2668
                      shift-left: w2667 -> [w2670]
                      n868 = Enqueue Element(queue=w2670, element=w2669) -> (queue out=w2671:refnum<queue>)  [unwired: 2 in, 2 out]
                    }
                  }
                  frame True {
                    n869 = for {